vi "UHR-Fleezers Control (host) - Avogadro v2.vi"() -> ()   [LabVIEW 2014] (continued)
          tunnel: [FALSE w2222] -> w2201
          frame False {
          }
          frame True {
            n1371 = local read "Green FB On/Off"() -> (w2223:bool)
            n1372 = Equal?(x=w2226, y=enum32{"Laser ON", "Laser OFF", "Interlace"}."Interlace") -> (x = y?=w2224:bool)
            n1373 = And(x=w2224, y=w2223) -> (x .and. y?=w2222:bool)
          }
        }
        n1374 = case shown="True" "Red Laser ON" {
          tunnel: "Laser interlacing mode" -> [_ w2219]
          tunnel: [enum32{"Laser ON", "Laser OFF", "Interlace"}."Laser OFF" ("Green laser mode") w2219] -> w2198
          tunnel: [FALSE w2215] -> w2197
          frame False {
          }
          frame True {
            n1375 = local read "Red FB On/Off"() -> (w2216:bool)
            n1376 = Equal?(x=w2219, y=enum32{"Laser ON", "Laser OFF", "Interlace"}."Interlace") -> (x = y?=w2217:bool)
            n1377 = And(x=w2217, y=w2216) -> (x .and. y?=w2215:bool)
          }
        }
        n1378 = case shown="True" "Blue Laser ON" {
          tunnel: "Laser interlacing mode" -> [_ w2210]
          tunnel: [enum32{"Laser ON", "Laser OFF", "Interlace"}."Laser OFF" ("Green laser mode") w2210] -> w2194
          tunnel: [FALSE w2208] -> w2193
          frame False {
          }
          frame True {
            n1379 = local read "Blue FB On/Off"() -> (w2209:bool)
            n1380 = Equal?(x=w2210, y=enum32{"Laser ON", "Laser OFF", "Interlace"}."Interlace") -> (x = y?=w2211:bool)
            n1381 = And(x=w2211, y=w2209) -> (x .and. y?=w2208:bool)
          }
        }
        n1382 = xnode "Read/Write Control"("FPGA VI Reference In"=w2192, "Operating Mode"=w2202, "Operating Mode 2"=w2202, "Green FB On/Off"=w2201, "Red Laser Operating Mode"=w2198, "RI Operating Mode 2"=w2198, "Red FB On/Off"=w2197, "BI Operating Mode (AO)"=w2194, "Blue Laser Operating Mode (D)"=w2194, "Blue FB On/Off"=w2193) -> ("error out"=w2203:errorcluster)  [unwired: 1 in, 1 out]
        n1383 = local read "Red FB On/Off"() -> (w2175:bool)
        n1384 = local read "Green FB On/Off"() -> (w2177:bool)
        n1385 = local read "Green Laser ON"() -> (w2176:bool)
        n1386 = local read "Red Laser ON"() -> (w2174:bool)
        n1387 = And(x=w2175, y=w2174) -> (x .and. y?=w2180:bool)
        n1388 = And(x=w2177, y=w2176) -> (x .and. y?=w2186:bool)
        n1389 = local read "Red laser intensity (V)"() -> (w2179:dbl)
        n1390 = local read "Red FB Setpoint (mV)"() -> (w2178:dbl)
        n1391 = local read "Green FB Setpoint (mV)"() -> (w2189:dbl)
        n1392 = local read "Green laser intensity (V)"() -> (w2191:dbl)
        n1393 = Multiply(x=w2179, y=1000.0) -> (x*y=w2183:dbl)
        n1394 = Subtract(x=w2178, y=5.0) -> (x-y=w2182:dbl)
        n1395 = Multiply(x=w2191, y=1000.0) -> (x*y=w2188:dbl)
        n1396 = Subtract(x=w2189, y=5.0) -> (x-y=w2187:dbl)
        n1397 = Less Or Equal?(x=w2183, y=w2182) -> (x <= y?=w2181:bool)
        n1398 = Less Or Equal?(x=w2188, y=w2187) -> (x <= y?=w2185:bool)
        n1399 = And(x=w2180, y=w2181) -> (x .and. y?=w2170:bool)
        n1400 = And(x=w2186, y=w2185) -> (x .and. y?=w2171:bool)
        n1401 = Or(x=w2171, y=w2170) -> (x .or. y?=w2169:bool)
        n1402 = case shown="True" w2169 {
          frame False {
            n1403 = local write "Laser Intensity Low (bugs to fix)"(FALSE ("Laser Intensity Low")) -> ()
          }
          frame True {
            n1404 = local write "Laser Intensity Low (bugs to fix)"(TRUE ("Laser Intensity Low")) -> ()
          }
        }
      }
      event "Invert laser interlacing", "RF BD 2 to green AOM": Value Change {
        n1405 = event-data() -> ()  [unwired: 7 out]
        n1406 = local read "RF BD 2 to green AOM"() -> (w2227:bool)
        n1407 = xnode "Read/Write Control"("FPGA VI Reference In"=w2228, "Invert GI"="Invert laser interlacing", "Invert GI 2"="Invert laser interlacing", "Invert RI"="Invert laser interlacing", "Invert RI 2"="Invert laser interlacing", "Invert BI (AO)"="Invert laser interlacing", "Invert BI (D)"="Invert laser interlacing", "RF synth bd controls green"=w2227) -> ("error out"=w2230:errorcluster)  [unwired: 1 in, 1 out]
      }
      event "Green FB Setpoint (mV)", "Green FB Gains", "Green FB On/Off", "Green Intensity % (FB OFF)", "Green int current ON count adj": Value Change {
        n1408 = event-data() -> ()  [unwired: 7 out]
        n1409 = local read "Green FB Setpoint (mV)"() -> (w2250:dbl)
        n1410 = Multiply(x=w2250, y=3.2767) -> (x*y=w2249:dbl)
        n1411 = local read "Green Intensity % (FB OFF)"() -> (w2253:dbl)
        n1412 = Multiply(x=w2253, y=655.35) -> (x*y=w2254:dbl)
        n1413 = To Unsigned Word Integer(number=w2254) -> (unsigned 16bit integer=w2252:u16)
        n1414 = local read "Green int current ON count adj"() -> (w2256:u32)
        n1415 = local read "Laser interlacing mode"() -> (w2247:enum32{"Laser ON", "Laser OFF", "Interlace"})
        n1416 = local read "Green FB Gains"() -> (w2244:T18)
        n1417 = local read "Green Laser ON"() -> (w2248:bool)
        n1418 = local read "Green FB On/Off"() -> (w2257:bool)
        n1419 = Equal?(x=w2247, y=enum32{"Laser ON", "Laser OFF", "Interlace"}."Interlace") -> (x = y?=w2245:bool)
        n1420 = Unbundle By Name(w2244) -> ("proportional gain (Kc)"=w2243:i16, "integral gain (Kc*Ts/Ti)"=w2242:i16, "derivative gain (Kc*Td/Ts)"=w2241:i16)
        n1421 = Compound Arithmetic op=AND(w2245, w2257, w2248) -> (w2231:bool)
        n1422 = local read "Green FB Setpoint (mV)"() -> (w2235:dbl)
        n1423 = local read "Green laser intensity (V)"() -> (w2238:dbl)
        n1424 = xnode "Read/Write Control"("FPGA VI Reference In"=w2240, "Green FB Setpoint"=w2249, "Green FB On/Off"=w2231, "Current Out"=w2252, "Green int current ON count adj"=w2256, "P3"=w2243, "I3"=w2242, "D3"=w2241) -> ("error out"=w2258:errorcluster)  [unwired: 1 in, 1 out]
        n1425 = Multiply(x=w2238, y=1000.0) -> (x*y=w2234:dbl)
        n1426 = Subtract(x=w2235, y=5.0) -> (x-y=w2233:dbl)
        n1427 = Less Or Equal?(x=w2234, y=w2233) -> (x <= y?=w2232:bool)
        n1428 = And(x=w2231, y=w2232) -> (x .and. y?=w2239:bool)
        n1429 = case shown="True" w2239 {
          frame False {
            n1430 = local write "Laser Intensity Low (bugs to fix)"(FALSE ("Laser Intensity Low")) -> ()
          }
          frame True {
            n1431 = local write "Laser Intensity Low (bugs to fix)"(TRUE ("Laser Intensity Low")) -> ()
          }
        }
      }
      event "Blue FB Setpoint (mV)", "Blue FB Gains", "Blue FB On/Off", "Blue Intensity % (FB OFF)", "Blue int AO ON count adjust": Value Change {
        # "Triggers blue laser serial command"
        # "16 bit analog out"
        n1432 = event-data() -> ()  [unwired: 7 out]
        n1433 = Multiply(x="Blue FB Setpoint (mV)", y=3.2767) -> (x*y=w2278:dbl)
        n1434 = Multiply(x="Blue Intensity % (FB OFF)", y=0.8) -> (x*y=w2261:dbl)
        n1435 = Number To Decimal String(number=w2261) -> (decimal integer string=w2262:string)  [unwired: 1 in]
        n1436 = Multiply(x="Blue Intensity % (FB OFF)", y=655.35) -> (x*y=w2281:dbl)
        n1437 = local write "Blue Laser Power (mW)\n(Constant Power Mode)"(w2262) -> ()
        n1438 = To Unsigned Word Integer(number=w2281) -> (unsigned 16bit integer=w2280:u16)
        n1439 = local read "Laser interlacing mode"() -> (w2276:enum32{"Laser ON", "Laser OFF", "Interlace"})
        n1440 = Unbundle By Name("Blue FB Gains") -> ("proportional gain (Kc)"=w2273:i16, "integral gain (Kc*Ts/Ti)"=w2272:i16, "derivative gain (Kc*Td/Ts)"=w2271:i16)
        n1441 = local read "Blue Laser ON"() -> (w2266:bool)
        n1442 = Equal?(x=w2276, y=enum32{"Laser ON", "Laser OFF", "Interlace"}."Interlace") -> (x = y?=w2274:bool)
        n1443 = Compound Arithmetic op=AND(w2274, "Blue FB On/Off", w2266) -> (w2277:bool)
        n1444 = xnode "Read/Write Control"("FPGA VI Reference In"=w2265, "Blue FB Setpoint"=w2278, "Blue FB On/Off"=w2277, "BI Current Out"=w2280, "Blue current ON count adj (AO)"="Blue int AO ON count adjust", "P5"=w2273, "I5"=w2272, "D5"=w2271) -> ("error out"=w2283:errorcluster)  [unwired: 1 in, 1 out]
      }
      event "Red FB Setpoint (mV)", "Red FB Gains", "Red FB On/Off", "Red Intensity % (FB OFF)": Value Change {
        n1445 = event-data() -> ()  [unwired: 7 out]
        n1446 = local read "Red FB Setpoint (mV)"() -> (w2304:dbl)
        n1447 = Multiply(x=w2304, y=3.2767) -> (x*y=w2303:dbl)
        n1448 = local read "Red Intensity % (FB OFF)"() -> (w2294:dbl)
        n1449 = Multiply(x=w2294, y=655.35) -> (x*y=w2307:dbl)
        n1450 = To Unsigned Word Integer(number=w2307) -> (unsigned 16bit integer=w2306:u16)
        n1451 = local read "Laser interlacing mode"() -> (w2301:enum32{"Laser ON", "Laser OFF", "Interlace"})
        n1452 = local read "Red FB Gains"() -> (w2298:T18)
        n1453 = local read "Red Laser ON"() -> (w2302:bool)
        n1454 = local read "Red FB On/Off"() -> (w2309:bool)
        n1455 = Equal?(x=w2301, y=enum32{"Laser ON", "Laser OFF", "Interlace"}."Interlace") -> (x = y?=w2299:bool)
        n1456 = Unbundle By Name(w2298) -> ("proportional gain (Kc)"=w2297:i16, "integral gain (Kc*Ts/Ti)"=w2296:i16, "derivative gain (Kc*Td/Ts)"=w2295:i16)
        n1457 = Compound Arithmetic op=AND(w2299, w2309, w2302) -> (w2286:bool)
        n1458 = local read "Red laser intensity (V)"() -> (w2285:dbl)
        n1459 = local read "Red FB Setpoint (mV)"() -> (w2284:dbl)
        n1460 = xnode "Read/Write Control"("FPGA VI Reference In"=w2293, "Red FB Setpoint"=w2303, "Red FB On/Off"=w2286, "RI Current Out"=w2306, "P4"=w2297, "I4"=w2296, "D4"=w2295) -> ("error out"=w2310:errorcluster)  [unwired: 1 in, 1 out]
        n1461 = Multiply(x=w2285, y=1000.0) -> (x*y=w2290:dbl)
        n1462 = Subtract(x=w2284, y=5.0) -> (x-y=w2289:dbl)
        n1463 = Less Or Equal?(x=w2290, y=w2289) -> (x <= y?=w2288:bool)
        n1464 = And(x=w2286, y=w2288) -> (x .and. y?=w2287:bool)
        n1465 = case shown="False" w2287 {
          frame False {
            n1466 = local write "Laser Intensity Low (bugs to fix)"(FALSE ("Laser Intensity Low")) -> ()
          }
          frame True {
            n1467 = local write "Laser Intensity Low (bugs to fix)"(TRUE ("Laser Intensity Low")) -> ()
          }
        }
      }
      event "+ phase (APD 1 Gate)", "- phase (APD 1 Gate)", "+ phase (APD 2 Gate)", "- phase (APD 2 Gate)", "+ phase (APD 3 Gate)", "- phase (APD 3 Gate)", "+ phase (APD Acq)", "- phase (APD Acq)": Value Change {
        n1468 = event-data() -> ()  [unwired: 7 out]
        n1469 = local read "Phase Adj. (APD 1 Gate)"() -> (w2333:i16)
        n1470 = Or(x="- phase (APD 1 Gate)", y="+ phase (APD 1 Gate)") -> (x .or. y?=w2335:bool)
        n1471 = Negate(x=w2333) -> (-x=w2340:i16)
        n1472 = Select(t=w2340, s="+ phase (APD 1 Gate)", f=w2333) -> (s? t:f=w2339:i16)
        n1473 = local read "Phase Adj. (APD 2 Gate)"() -> (w2330:i16)
        n1474 = Or(x="- phase (APD 2 Gate)", y="+ phase (APD 2 Gate)") -> (x .or. y?=w2328:bool)
        n1475 = Negate(x=w2330) -> (-x=w2332:i16)
        n1476 = Select(t=w2332, s="+ phase (APD 2 Gate)", f=w2330) -> (s? t:f=w2329:i16)
        n1477 = Negate(x="Phase Adj. (APD 3 Gate)") -> (-x=w2327:i16)
        n1478 = Or(x="- phase (APD 3 Gate)", y="+ phase (APD 3 Gate)") -> (x .or. y?=w2323:bool)
        n1479 = Select(t=w2327, s="+ phase (APD 3 Gate)", f="Phase Adj. (APD 3 Gate)") -> (s? t:f=w2324:i16)
        n1480 = local read "Phase Adj. (APD Acq)"() -> (w2321:i16)
        n1481 = Or(x="- phase (APD Acq)", y="+ phase (APD Acq)") -> (x .or. y?=w2319:bool)
        n1482 = Negate(x=w2321) -> (-x=w2322:i16)
        n1483 = Select(t=w2322, s="+ phase (APD Acq)", f=w2321) -> (s? t:f=w2320:i16)
        n1484 = xnode "Read/Write Control"("FPGA VI Reference In"=w2313, "Phase count adjustment (APD 1 Gate)"=w2339, "Phase count adjustment (APD 2 Gate)"=w2329, "Phase count adjustment (APD 3 Gate)"=w2324, "Phase Count Adjustment (APD Acq)"=w2320) -> ("FPGA VI Reference Out"=w2337:T40, "error out"=w2338:errorcluster)  [unwired: 1 in]
        n1485 = xnode "Read/Write Control"("FPGA VI Reference In"=w2337, "error in"=w2338, "+ phase (APD 1 Gate)"=w2335, "+ phase (APD 2 Gate)"=w2328, "+ phase (APD 3 Gate)"=w2323, "+ phase (APD Acq)"=w2319) -> ("error out"=w2336:errorcluster)  [unwired: 1 out]
      }
      event "Invert APD Gate", "APD Gate ON Count", "APD Gate OFF Count", "APD Gate", "APD Integration Time (s)", "APD AO Scale Factor", "Duty Frequency (ON 1/N cycles)", "Interlace ON count", "Interlace OFF count": Value Change {
        n1486 = event-data() -> ()  [unwired: 7 out]
        n1487 = Add(x="Interlace ON count", y="Interlace OFF count") -> (x+y=w2347:u16)
        n1488 = Add(x="APD Gate ON Count", y="APD Gate OFF Count") -> (x+y=w2358:u16)
        n1489 = Multiply(x="Duty Frequency (ON 1/N cycles)", y=w2347) -> (x*y=w2343:u16)
        "Green AI Count" <- w2343
        "Red AI Count" <- w2343
        "Blue AI Count" <- w2343
        n1490 = Subtract(x=w2343, y="Interlace ON count") -> (x-y=w2346:u16)
        n1491 = Multiply(x=w2358, y="Duty Frequency (ON 1/N cycles)") -> (x*y=w2357:u16)
        n1492 = Subtract(x=w2357, y="APD Gate ON Count") -> (x-y=w2356:u16)
        n1493 = local read "DMA Update Period (s)"() -> (w2359:dbl)
        n1494 = Multiply(x="APD Integration Time (s)", y=40000000.0) -> (x*y=w2363:dbl)
        n1495 = Reciprocal(x="APD Integration Time (s)") -> (1/x=→"APD Acq Rate (Hz)":dbl)
        n1496 = To Unsigned Long Integer(number=w2363) -> (unsigned 32bit integer=w2349:u32)
        "APD Int. Count" <- w2349
        n1497 = local read "Number of APDs"() -> (w2342:u8)
        n1498 = Divide(x=w2359, y="APD Integration Time (s)") -> (x/y=w2361:dbl)
        n1499 = Multiply(x=w2342, y=w2361) -> (x*y=w2360:dbl)
        n1500 = local write "APD Samples/FIFO Acq."(w2361) -> ()
        n1501 = local write "APD Elements/DMA read"(w2360) -> ()
        n1502 = xnode "Read/Write Control"("FPGA VI Reference In"=w2341, "Invert APD Gate"="Invert APD Gate", "APD Gate ON Count"="APD Gate ON Count", "APD Gate OFF Count"=w2356, "APD Acq Rate Count"=w2349, "APD Gate Operating Mode"="APD Gate", "APD AO scale factor"="APD AO Scale Factor", "Green interlace ON count 2"="Interlace ON count", "Green interlace OFF count 2"=w2346, "Green FB Count"=w2343, "Red interlace ON count"="Interlace ON count", "Red interlace OFF count"="Interlace OFF count", "Blue ON count (AO)"="Interlace ON count", "Blue OFF count (AO)"="Interlace OFF count", "Blue interlace OFF count (D)"="Interlace OFF count", "Blue interlace ON count (D)"="Interlace ON count") -> ("error out"=w2365:errorcluster)  [unwired: 1 in, 1 out]
      }
      event "Neg. TTrig FPGA": Value Change {
        n1503 = event-data() -> ()  [unwired: 7 out]
        n1504 = xnode "Read/Write Control"("FPGA VI Reference In"=w2366, "TTrig Negate Pos"="Neg. TTrig FPGA") -> ()  [unwired: 1 in, 2 out]
      }
      event "Test ttrig": Value Change {
        n1505 = event-data() -> ()  [unwired: 7 out]
        n1506 = xnode "Read/Write Control"("FPGA VI Reference In"=w2368, "TTrig?"=TRUE) -> ("error out"=w2370:errorcluster)  [unwired: 1 in, 1 out]
      }
      event "Number of F/B Scans (AOD)", "Scan Speed (nm/s)", "Scan BD", "Initial delta (MHz)", "Step Size (nm)", "Scan Range (nm)": Value Change {
        w2434 = 123.0  # AOM cal (nm/MHz)
        n1507 = event-data() -> ()  [unwired: 7 out]
        n1508 = local read "BD 1 Frequency 1 (MHz)"() -> (w2417:dbl)
        n1509 = local read "AOM X Cal (nm/MHz)"() -> (w2409:dbl)
        n1510 = local read "X RF Frequency Limits (MHz)"() -> (w2421:T26)
        n1511 = local read "Y RF Frequency Limits (MHz)"() -> (w2418:T26)
        n1512 = local read "BD 2 Frequency 1 (MHz)"() -> (w2423:dbl)
        n1513 = Negate(x="Scan Range (nm)") -> (-x=w2387:dbl)
        n1514 = Divide(x=w2387, y=w2409) -> (x/y=w2391:dbl)
        n1515 = Select(t=w2421, s="Scan BD", f=w2418) -> (s? t:f=w2420:T26)
        n1516 = Select(t=w2417, s="Scan BD", f=w2423) -> (s? t:f=w2422:dbl)
        n1517 = Unbundle By Name(w2420) -> ("Maximum"=w2429:dbl, "Minimum"=w2428:dbl)
        n1518 = Add(x=w2391, y=w2422) -> (x+y=w2426:dbl)
        n1519 = Divide(x=w2387, y="Step Size (nm)") -> (x/y=w2406:dbl)
        n1520 = Divide(x="Step Size (nm)", y=w2409) -> (x/y=w2415:dbl)
        n1521 = Absolute Value(x=w2406) -> (abs(x)=w2390:dbl)
        n1522 = Sign(1:w2387) -> (0:w2388:dbl)
        n1523 = In Range and Coerce(upper limit=w2429, x=w2426, lower limit=w2428) -> (coerced(x)=w2425:dbl, In Range?=w2427:bool)
        n1524 = To Unsigned Quad Integer(1:w2390) -> (0:w2405:u64)
        "Scan steps (AOD)" <- w2405
        n1525 = call "IR AOM freq to word.vi"("Frequency In (MHz)"=w2415) -> ("Frequency Word Out (double)"=w2412:dbl)
        n1526 = Multiply(x=w2388, y=w2412) -> (x*y=w2389:dbl)
        n1527 = Subtract(x=w2426, y=w2425) -> (x-y=w2424:dbl)
        n1528 = To Quad Integer(1:w2389) -> (0:w2411:i64)
        "Incr. int (AOD)" <- w2411
        n1529 = Subtract(x=w2391, y=w2424) -> (x-y=w2410:dbl)
        "Scan Range (MHz)" <- w2410
        n1530 = Select(t=w2391, s=w2427, f=w2410) -> (s? t:f=w2430:dbl)
        n1531 = Multiply(x=w2410, y=w2409) -> (x*y=w2408:dbl)
        n1532 = Decrement(x=w2405) -> (x-1=w2458:u64)
        n1533 = Negate(x=w2408) -> (-x=w2404:dbl)
        n1534 = local write "Scan Range (nm)"(w2404) -> ()
        n1535 = Divide(x=w2430, y=w2458) -> (x/y=w2414:dbl)
        "Scan Increment (MHz)" <- w2414
        n1536 = call "IR AOM freq to word.vi"("Frequency In (MHz)"=w2414) -> ("Frequency Word Out (double)"=w2413:dbl)
        n1537 = Divide(x="Step Size (nm)", y="Scan Speed (nm/s)") -> (x/y=w2401:dbl)
        n1538 = To Quad Integer(1:w2413) -> ()  [unwired: 1 out]
        n1539 = local read "Number Interlace Sets"() -> (w2385:u8)
        n1540 = local read "AI Count (ticks)"() -> (w2386:u16)
        n1541 = local read "Total Counts (ticks)"() -> (w2384:u16)
        n1542 = local read "# Samples/trap"() -> (w2416:u32)
        n1543 = Multiply(x=w2386, y=w2385) -> (x*y=w2383:u16)
        n1544 = Divide(x=w2384, y=w2383) -> (x/y=w2382:dbl)
        n1545 = Select(t=w2417, s="Scan BD", f=w2423) -> (s? t:f=w2455:dbl)
        "Initial freq. (MHz)" <- w2455
        n1546 = Add(x=w2430, y=w2455) -> (x+y=→"Final freq. (MHz)":dbl)
        n1547 = Divide(x=w2384, y=40000000.0) -> (x/y=w2400:dbl)
        n1548 = Divide(x=w2401, y=w2400) -> (x/y=w2399:dbl)
        n1549 = To Unsigned Quad Integer(1:w2399) -> (0:w2374:u64)
        n1550 = Quotient & Remainder(x=w2374, y=u64 2) -> (x-y*floor(x/y)=w2378:u64)  [unwired: 1 out]
        n1551 = Equal?(x=w2378, y=u64 0) -> (x = y?=w2376:bool)
        n1552 = Decrement(x=w2374) -> (x-1=w2375:u64)
        n1553 = Select(t=w2374, s=w2376, f=w2375) -> (s? t:f=w2373:u64)
        "Cycles/step (AOD)" <- w2373
        n1554 = xnode "Read/Write Control"("FPGA VI Reference In"=w2372, "Scan steps"=w2405, "Number of scans"="Number of F/B Scans (AOD)", "Cycles per step"=w2373, "Scan freq.  increment"=w2411, "Scan BD"="Scan BD") -> ("error out"=w2464:errorcluster)  [unwired: 1 in, 1 out]
        n1555 = Multiply(x=w2405, y=w2373) -> (x*y=w2459:u64)
        n1556 = Multiply(x=w2459, y=u64 2) -> (x*y=w2381:u64)
        n1557 = Multiply(x=w2382, y=w2381) -> (x*y=w2380:dbl)
        "Data points/scan (f/b)" <- w2380
        n1558 = Multiply(x=w2380, y="Number of F/B Scans (AOD)") -> (x*y=w2462:dbl)
        "Data points/scans" <- w2462
        n1559 = Divide(x=w2462, y=w2416) -> (x/y=→"N sets should be saved":dbl)
        n1560 = Multiply(x=w2459, y=w2400) -> (x*y=w2398:dbl)
        "Time/Scan (s) (AOD)" <- w2398
        n1561 = Select(t=w2430, s="Scan BD", f=0.0) -> (s? t:f=w2456:dbl)
        n1562 = Select(t=0.0, s="Scan BD", f=w2430) -> (s? t:f=w2452:dbl)
        n1563 = local read "BD 2 Frequency 2 (MHz)"() -> (w2448:dbl)
        n1564 = local read "BD 1 Frequency 2 (MHz)"() -> (w2451:dbl)
        n1565 = Add(x=w2452, y=w2423) -> (x+y=w2449:dbl)
        n1566 = Add(x=w2417, y=w2456) -> (x+y=w2450:dbl)
        n1567 = Multiply(x=w2398, y=2.0) -> (x*y=w2397:dbl)
        n1568 = Multiply(x=w2397, y="Number of F/B Scans (AOD)") -> (x*y=w2394:dbl)
        n1569 = Divide(x=w2394, y=60.0) -> (x/y=→"Time to Finish All (min)":dbl)
        n1570 = Add(x="Trap 2 Bead Size (nm)", y="Trap 1 Bead Size (nm)") -> (x+y=w2438:dbl)
        n1571 = Divide(x=w2438, y=2.0) -> (x/y=w2432:dbl)
        n1572 = local read "Initial delta (MHz)"() -> (w2435:dbl)
        n1573 = Subtract(x=w2449, y=w2448) -> (x-y=w2446:dbl)
        n1574 = Subtract(x=w2450, y=w2451) -> (x-y=w2447:dbl)
        n1575 = Square(x=w2446) -> (x^2=w2445:dbl)
        n1576 = Square(x=w2447) -> (x^2=w2444:dbl)
        n1577 = Add(x=w2444, y=w2445) -> (x+y=w2443:dbl)
        n1578 = Square Root(x=w2443) -> (sqrt(x)=w2442:dbl)
        "Final delta (MHz)" <- w2442
        n1579 = Multiply(x=w2434, y=w2442) -> (x*y=w2441:dbl)
        n1580 = Multiply(x=w2435, y=w2434) -> (x*y=w2433:dbl)
        n1581 = Subtract(x=w2433, y=w2432) -> (x-y=→"Initial sep (nm)":dbl)
        n1582 = Subtract(x=w2441, y=w2432) -> (x-y=→"Final sep (nm)":dbl)
      }
      event "Swap F1 and F2", "RF amplitude switch delay": Value Change {
        n1583 = event-data() -> ()  [unwired: 7 out]
        n1584 = local read "RF amplitude switch delay"() -> (w2466:u16)
        n1585 = local read "Swap F1 and F2"() -> (w2467:bool)
        n1586 = xnode "Read/Write Control"("FPGA VI Reference In"=w2465, "Swap F1 and F2"=w2467, "Amp switch delay"=w2466) -> ("error out"=w2468:errorcluster)  [unwired: 1 in, 1 out]
      }
      event "Scan steps (MCL)", "Number of scans (MCL)", "Scan Range (V)\n(of steps)", "2D or 1D Scan", "N APD Samp/step", "Fast Scan Dir", "Continuous MCL Scanning", "Scan lines (y)": Value Change {
        w2471 = 32767.0 ("y")
        n1587 = event-data() -> ()  [unwired: 7 out]
        n1588 = Select(t="Scan lines (y)", s="2D or 1D Scan", f="Number of scans (MCL)") -> (s? t:f=w2476:u64)
        n1589 = Decrement(x="Scan steps (MCL)") -> (x-1=w2492:u64)
        n1590 = Divide(x="Scan Range (V)\n(of steps)", y=w2492) -> (x/y=w2491:dbl)
        "Desired Scan Incr (V)" <- w2491
        n1591 = local read "APD Integration Time (s)"() -> (w2484:dbl)
        n1592 = Multiply(x=w2491, y=w2471) -> (x*y=w2500:dbl)
        n1593 = Divide(x=w2500, y=10.0) -> (x/y=w2490:dbl)
        "Desired incr (int)" <- w2490
        n1594 = local read "Update Count (MCL)"() -> (w2496:u32)
        n1595 = Round Toward -Infinity(1:w2490) -> (0:w2499:dbl)
        n1596 = To Word Integer(number=w2499) -> (16bit integer=w2474:i16)
        "Actual Incr. int (MCL)" <- w2474
        n1597 = Multiply(x=w2484, y=40000000.0) -> (x*y=w2497:dbl)
        n1598 = Divide(x=w2497, y=w2496) -> (x/y=w2495:dbl)
        n1599 = Multiply(x=i16 10, y=w2474) -> (x*y=w2472:i16)
        n1600 = Multiply(x="N APD Samp/step", y=w2495) -> (x*y=w2494:dbl)
        "Cycles/step (MCL)" <- w2494
        n1601 = Divide(x=w2472, y=w2471) -> (x/y=→"Actual MCL Inc (V)":dbl)
        n1602 = Multiply(x="N APD Samp/step", y="Scan steps (MCL)") -> (x*y=w2486:dbl)
        n1603 = local read "APD Samples/FIFO Acq."() -> (w2483:dbl)
        n1604 = Multiply(x=w2486, y=u64 2) -> (x*y=w2485:dbl)
        "Data points/scan (f+b)" <- w2485
        n1605 = Multiply(x=w2485, y=w2476) -> (x*y=w2503:dbl)
        "Data points/scans (MCL)" <- w2503
        n1606 = Multiply(x=w2484, y=w2485) -> (x*y=w2477:dbl)
        "Time/f+b scan (s) (MCL)" <- w2477
        n1607 = Divide(x=w2503, y=w2483) -> (x/y=→"N sets should be saved (MCL)":dbl)
        n1608 = Multiply(x=w2477, y=w2476) -> (x*y=→"Total Time (s)":dbl)
        n1609 = Not(x="Fast Scan Dir") -> (.not. x?=w2481:bool)
        n1610 = xnode "Read/Write Control"("FPGA VI Reference In"=w2469, "Scan steps (MCL)"="Scan steps (MCL)", "Number of scans (MCL)"=w2476, "Cycles per step (MCL)"=w2494, "Scan freq.  increment (MCL)"=w2474, "1D or 2D Scan?"="2D or 1D Scan", "MCL Scan Axis"=w2481, "Cont. Scan (MCL)"="Continuous MCL Scanning") -> ("error out"=w2505:errorcluster)  [unwired: 1 in, 1 out]
      }
      event "Read Cal": Value Change {
        w2528 = T53."big-endian, network order" ("byte order (0:big-endian, network order)")
        n1611 = event-data() -> ()  [unwired: 7 out]
        n1612 = local read "Save file name"() -> (w2553:path)
        n1613 = Strip Path(path=w2553) -> (stripped path=w2552:path)  [unwired: 1 out]
        n1614 = Path To String(path=w2552) -> (string=w2545:string)
        n1615 = Concatenate Strings(w2545, "\\current.cal" ("string")) -> (w2550:string)
        n1616 = String To Path(string=w2550) -> (path=w2549:path)
        n1617 = Concatenate Strings(w2545, "\\current.off" ("string")) -> (w2543:string)
        n1618 = Open/Create/Replace File(file path (use dialog)=w2549, operation (0:open)=T52."open", access (0:read/write)=enum16{"read/write", "read-only", "write-only"}."read-only") -> (refnum out=w2556:refnum<file>, error out=w2548:errorcluster)  [unwired: 1 in, 3 out]
        n1619 = Deny Access(4:w2548, 7:w2556) -> (0:w2529:errorcluster, 3:w2524:refnum<file>)  [unwired: 1 out]
        n1620 = String To Path(string=w2543) -> (path=w2540:path)
        n1621 = local write "Read Cal"(FALSE ("Read Cal")) -> ()
        n1622 = Open/Create/Replace File(file path (use dialog)=w2540, operation (0:open)=T52."open", access (0:read/write)=enum16{"read/write", "read-only", "write-only"}."read-only") -> (refnum out=w2539:refnum<file>)  [unwired: 1 in, 4 out]
        n1623 = Deny Access(7:w2539) -> (3:w2538:refnum<file>)  [unwired: 1 in, 2 out]
        n1624 = Read from Binary File(5:0.0, 9:w2528, 10:-1 ("count (1)"), 11:w2538) -> (2:w2506:dbl[], 3:w2535:refnum<file>)  [unwired: 1 in, 3 out]
        "Raw offsets" <- w2506
        n1625 = local read "Multiple-MCL offset?"() -> (w2507:bool)
        n1626 = Close File(refnum=w2535) -> ()  [unwired: 1 in, 2 out]
        n1627 = case shown="True" w2507 {
          tunnel: w2506 -> [w2561 w2568]
          tunnel: [w2558 w2566] -> w2533
          tunnel: [w2557 w2565] -> w2532
          frame False {
            # "If not doing multiple offset, same calculation as before"
            n1628 = Decimate 1D Array(w2561) -> (w2558:dbl[], w2557:dbl[])
            n1629 = Bundle By Name(cluster="Two Trap Offset Values", "Trap 1X offset"=w2558, "Trap 2X offset"=w2557) -> (w2559:T31)
            n1630 = local write "Two Trap Offset Values"(w2559) -> ()
          }
          frame True {
            w2563 = 0.0
            # "When doing multiple offset: separate data to different scans, make array of clusters of 1x,1y,2x,2y,3x,3y arrays"
            n1631 = local read "MCL offset scanning range (V)"() -> (w2569:T4)
            n1632 = local read "Offset file step size"() -> (w2567:dbl)
            n1633 = Build Array(w2563, w2563, w2563, w2563, w2563, w2563) -> (w2562:dbl[])
            n1634 = call "generate multiple MCL offset.vi"("Offset array"=w2568, "offset file step size"=w2567, "MCL offset scanning range (V)"=w2569, "Corrections"=w2562) -> ("B_X mean out"=w2565:dbl[], "A_X mean out"=w2566:dbl[], "Output array"=→"Multi-MCL offset array":T30)
          }
        }
        n1635 = Build Array("T1 calibration", "T2 calibration", "T3 calibration") -> (w2520:T55)
        n1636 = for {
          N: 3 ("count (1)") -> [_]
          tunnel: w2528 -> [w2587]
          shift-right: [w2585] -> w2526
          shift-left: w2529 -> [w2588]
          shift-right: [w2584] -> w2525
          shift-left: w2524 -> [w2583]
          tunnel: w2520 -> [w2582] mode=indexing
          tunnel: [w2576] -> w2519 mode=indexing
          i -> [w2577]
          w2571 = 1000.0
          n1637 = Read from Binary File(5:0.0, 8:w2588, 9:w2587, 10:6 ("count (1)"), 11:w2583) -> (0:w2585:errorcluster, 2:w2590:dbl[], 3:w2584:refnum<file>)  [unwired: 2 out]
          n1638 = Array To Cluster(array=w2590) -> (cluster=w2581:T56)
          n1639 = Unbundle(w2581) -> ("[0]"=w2580:dbl, "[1]"=w2579:dbl, "[2]"=w2573:dbl, "[3]"=w2578:dbl, "[4]"=w2572:dbl, "[5]"=w2575:dbl)
          n1640 = Multiply(x=w2572, y=w2571) -> (x*y=w2570:dbl)
          n1641 = Multiply(x=w2571, y=w2575) -> (x*y=w2574:dbl)
          n1642 = Bundle By Name(cluster=w2582, "alpha_x (nm/V)"=w2580, "alpha_y (nm/V)"=w2579, "kappa_x (pN/nm)"=w2573, "kappa_y (pN/nm)"=w2578, "offset_x (mV)"=w2570, "offset_y (mV)"=w2574) -> (w2576:T12)
          n1643 = case shown="2" w2577 {
            tunnel: w2576 -> [w2591 w2592 w2593]
            frame 0, Default {
              n1644 = local write "T1 calibration"(w2591) -> ()
            }
            frame 1 {
              n1645 = local write "T2 calibration"(w2592) -> ()
            }
            frame 2 {
              n1646 = local write "T3 calibration"(w2593) -> ()
            }
          }
        }
        n1647 = Index Array(array=w2519, index=1) -> (element=w2516:T12)
        n1648 = Index Array(array=w2519, index=0) -> (element=w2515:T12)
        n1649 = Unbundle By Name(w2516) -> ("alpha_x (nm/V)"=w2514:dbl, "kappa_x (pN/nm)"=w2513:dbl)
        n1650 = Unbundle By Name(w2515) -> ("alpha_x (nm/V)"=w2512:dbl, "kappa_x (pN/nm)"=w2511:dbl)
        n1651 = Close File(refnum=w2525, error in=w2526) -> (error out=→"Read cal error":errorcluster)  [unwired: 1 out]
        n1652 = Multiply(x=w2514, y=w2513) -> (x*y=w2510:dbl)
        n1653 = Multiply(x=w2512, y=w2511) -> (x*y=w2509:dbl)
        n1654 = Divide(x=w2510, y=w2509) -> (x/y=w2508:dbl)
        n1655 = property on="B factor" class="DigNum (strict)"("Val(Sgnl)"=w2508) -> ()  [unwired: 2 in, 2 out]
        n1656 = Multiply(x=w2532, y=w2508) -> (x*y=w2534:dbl[])
        n1657 = Subtract(x=w2533, y=w2534) -> (x-y=w2530:dbl[])
        n1658 = case shown="True" "Auto read offset correction" {
          tunnel: w2530 -> [_ w2594]
          frame False {
          }
          frame True {
            n1659 = property on="Setpoint offset\ncorrection values" class="Arr (strict)"("Val(Sgnl)"=w2594) -> ()  [unwired: 2 in, 2 out]
          }
        }
      }
      event "Abort MCL Scan": Value Change {
        n1660 = event-data() -> ()  [unwired: 7 out]
        n1661 = local write "MCL Scanning"(FALSE ("MCL Scanning")) -> ()
        n1662 = xnode "Read/Write Control"("FPGA VI Reference In"=w2595, "Abort scan (MCL)"="Abort MCL Scan") -> ("error out"=w2598:errorcluster)  [unwired: 1 in, 1 out]
      }
      event "Update Count (MCL)": Value Change {
        n1663 = event-data() -> ()  [unwired: 7 out]
        n1664 = xnode "Read/Write Control"("FPGA VI Reference In"=w2599, "MCL count"="Update Count (MCL)") -> ("error out"=w2601:errorcluster)  [unwired: 1 in, 1 out]
      }
      event "+ phase (MCL)", "- phase (MCL)": Value Change {
        n1665 = event-data() -> ()  [unwired: 7 out]
        n1666 = Or(x="- phase (MCL)", y="+ phase (MCL)") -> (x .or. y?=w2605:bool)
        n1667 = Negate(x="Phase adjust (MCL)") -> (-x=w2611:i16)
        n1668 = Select(t=w2611, s="+ phase (MCL)", f="Phase adjust (MCL)") -> (s? t:f=w2609:i16)
        n1669 = xnode "Read/Write Control"("FPGA VI Reference In"=w2602, "Phase count adjustment (MCL)"=w2609) -> ("FPGA VI Reference Out"=w2606:T40, "error out"=w2607:errorcluster)  [unwired: 1 in]
        n1670 = xnode "Read/Write Control"("FPGA VI Reference In"=w2606, "error in"=w2607, "+ phase (MCL)"=w2605) -> ("error out"=w2604:errorcluster)  [unwired: 1 out]
      }
      event "Abort AOD Scan": Value Change {
        n1671 = event-data() -> ()  [unwired: 7 out]
        n1672 = xnode "Read/Write Control"("FPGA VI Reference In"=w2612, "Abort scan"="Abort AOD Scan") -> ("error out"=w2614:errorcluster)  [unwired: 1 in, 1 out]
      }
      event "Continuous AOD Scanning": Value Change {
        n1673 = event-data() -> ()  [unwired: 7 out]
        n1674 = xnode "Read/Write Control"("FPGA VI Reference In"=w2615, "Cont. Scan"="Continuous AOD Scanning") -> ("error out"=w2617:errorcluster)  [unwired: 1 in, 1 out]
      }
      event "Index": Value Change {
        n1675 = event-data() -> ()  [unwired: 7 out]
        n1676 = call "Create new save file.vi"("Insert"="", "Ext"=".dat" ("string"), "Index In"="Index") -> ("Path Out"=→"Save file name":path, "Index Out"=w2618:dbl)
        "Save index" <- w2618
        n1677 = local write "Index"(w2618) -> ()
      }
      event "AO1", "AO2": Value Change {
        w2632 = 10.0 ("y")
        w2631 = 32767.0 ("y")
        n1678 = event-data() -> ()  [unwired: 7 out]
        n1679 = local read "AO2"() -> (w2630:dbl)
        n1680 = local read "AO1"() -> (w2627:dbl)
        n1681 = Multiply(x=w2627, y=w2631) -> (x*y=w2626:dbl)
        n1682 = Multiply(x=w2630, y=w2631) -> (x*y=w2629:dbl)
        n1683 = Divide(x=w2626, y=w2632) -> (x/y=w2625:dbl)
        n1684 = Divide(x=w2629, y=w2632) -> (x/y=w2628:dbl)
        n1685 = To Word Integer(number=w2625) -> (16bit integer=w2633:i16)
        n1686 = To Word Integer(number=w2628) -> (16bit integer=w2634:i16)
        n1687 = xnode "Read/Write Control"("FPGA VI Reference In"=w2623, "AO1 (Y)"=w2633, "AO2 (X)"=w2634) -> ("error out"=w2624:errorcluster)  [unwired: 1 in, 1 out]
      }
      event "Inject Pump 1": Value Change {
        n1688 = event-data() -> ()  [unwired: 7 out]
        n1689 = disable-structure shown="Disabled" {
          disable-tunnel: w2635 -> [w2636 _]
          frame Disabled {
            n1690 = local read "Use Harvard pumps\nfor beads (else Chemyx)"() -> (w2637:bool)
            n1691 = case shown="True" w2637 {
              tunnel: "Inject Pump 1" -> [w2641 w2682]
              tunnel: w2636 -> [_ w2683]
              frame False {
                n1692 = local read "Pump write delay (ms)"() -> (w2640:dbl)
                n1693 = local read "Chemyx Syringe Pump Serial Port"() -> (w2639:refnum<visa-resource-name>)
                n1694 = case shown="True" w2641 {
                  tunnel: w2640 -> [w2647 w2661]
                  tunnel: w2639 -> [w2644 w2660]
                  frame False {
                    n1695 = flat-sequence {
                      tunnel: w2644 -> [w2648]
                      tunnel: [w2648] -> w2645
                      tunnel: w2647 -> [_]
                      tunnel: [w2651] -> w2646
                      tunnel: w2645 -> [w2651]
                      tunnel: w2646 -> [w2652]
                      tunnel: [w2652] -> w2642
                      tunnel: [w2654] -> w2643
                      tunnel: w2642 -> [w2654]
                      tunnel: w2643 -> [w2656]
                      frame #0 {
                        n1696 = call "Write to pump.vi"("string"="enter pump1", "VISA resource name"=w2648) -> ()  [unwired: 1 out]
                      }
                      frame #1 {
                        n1697 = Wait (ms)(milliseconds to wait="Pump pause delay (ms)") -> ()  [unwired: 1 out]
                      }
                      frame #2 {
                        n1698 = call "Write to pump.vi"("string"="stop", "VISA resource name"=w2652) -> ()  [unwired: 1 out]
                      }
                      frame #3 {
                        n1699 = Wait (ms)(milliseconds to wait=u32 500) -> ()  [unwired: 1 out]
                      }
                      frame #4 {
                        n1700 = call "Write to pump.vi"("string"="stop", "VISA resource name"=w2656) -> ()  [unwired: 1 out]
                      }
                    }
                  }
                  frame True {
                    n1701 = flat-sequence {
                      tunnel: w2660 -> [w2670]
                      tunnel: w2661 -> [w2665]
                      tunnel: w2661 -> [w2672]
                      tunnel: w2660 -> [w2673]
                      tunnel: [w2673] -> w2658
                      tunnel: [w2675] -> w2659
                      tunnel: w2658 -> [w2675]
                      tunnel: w2659 -> [w2677]
                      frame #0 {
                        n1702 = local read "All Pump Parameters"() -> (w2664:T14)
                        n1703 = Unbundle By Name(w2664) -> ("Pump 1"=w2671:T57)
                        n1704 = call "Set pump parameters.vi"("Pump write delay (ms)"=w2665, "Volume (uL)"="Ch 1 Inject Volume (uL)", "Rate (uL/h)"="Ch 1 Inject Rate (ul/h)", "Units"=4.0, "Pump #"=1.0, "Pump Parameters In"=w2671, "VISA resource name"=w2670) -> ("Pump Parameters Out"=w2663:T57)  [unwired: 3 in]
                        n1705 = Bundle By Name(cluster=w2664, "Pump 1"=w2663) -> (w2662:T14)
                        n1706 = local write "All Pump Parameters"(w2662) -> ()
                      }
                      frame #1 {
                        n1707 = Wait (ms)(milliseconds to wait=w2672) -> ()  [unwired: 1 out]
                      }
                      frame #2 {
                        n1708 = call "Write to pump.vi"("string"="start", "VISA resource name"=w2673) -> ()  [unwired: 1 out]
                      }
                      frame #3 {
                        n1709 = Wait (ms)(milliseconds to wait=u32 500) -> ()  [unwired: 1 out]
                      }
                      frame #4 {
                        n1710 = call "Write to pump.vi"("string"="start", "VISA resource name"=w2677) -> ()  [unwired: 1 out]
                      }
                    }
                  }
                }
              }
              frame True {
                n1711 = case shown="False" w2682 {
                  tunnel: w2683 -> [w2695 w2705]
                  frame False {
                    n1712 = flat-sequence {
                      tunnel: w2695 -> [w2697]
                      frame #0 {
                        n1713 = local write "Flushing P1"(FALSE ("Flushing P1")) -> ()
                        n1714 = Concatenate Strings("stop" ("string"), "\r") -> (w2699:string)
                        n1715 = VISA Write(VISA resource name=w2697, write buffer=w2699) -> ()  [unwired: 1 in, 3 out]
                      }
                      frame #1 {
                        n1716 = property on="Clear Volume P1" class="Bool (strict)"("Val(Sgnl)"=TRUE ("Value (Signaling)")) -> ()  [unwired: 2 in, 2 out]
                      }
                    }
                  }
                  frame True {
                    n1717 = local read "Normal Flow Rate (ul/h) P1"() -> (w2703:dbl)
                    n1718 = Number To Decimal String(number=w2703) -> (decimal integer string=w2709:string)  [unwired: 1 in]
                    n1719 = Concatenate Strings("irate  " ("string"), w2709, " u/h" ("string"), "\r") -> (w2707:string)
                    n1720 = VISA Write(VISA resource name=w2705, write buffer=w2707) -> (VISA resource name out=w2704:refnum<visa-resource-name>)  [unwired: 1 in, 2 out]
                    n1721 = Concatenate Strings("irun" ("string"), "\r") -> (w2711:string)
                    n1722 = VISA Write(VISA resource name=w2704, write buffer=w2711) -> ()  [unwired: 1 in, 3 out]
                  }
                }
                n1723 = local read "Saving..."() -> (w2680:bool)
                n1724 = local read "Save Event Log?"() -> (w2679:bool)
                n1725 = And(x=w2680, y=w2679) -> (x .and. y?=w2681:bool)
                n1726 = case shown="True" w2681 {
                  tunnel: w2682 -> [_ w2693]
                  frame False {
                  }
                  frame True {
                    n1727 = local read "Normal Flow Rate (ul/h) P1"() -> (w2684:dbl)
                    n1728 = Number To Decimal String(number=w2684) -> (decimal integer string=w2685:string)  [unwired: 1 in]
                    n1729 = Concatenate Strings("on, flow rate", w2685) -> (w2687:string)
                    n1730 = Select(t=w2687, s=w2693, f="off") -> (s? t:f=w2689:string)
                    n1731 = local read "log file ref"() -> (w2694:refnum<file>)
                    n1732 = local read "Time (s)"() -> (w2688:dbl)
                    n1733 = Concatenate Strings("pump 1 ", w2689) -> (w2691:string)
                    n1734 = call "write to event log.vi"("log file ref"=w2694, "time"=w2688, "input string"=w2691) -> ()  [unwired: 8 in]
                  }
                }
              }
            }
          }
          frame Enabled {
          }
        }
      }
      event "Shunt 1": Value Change {
        n1735 = event-data() -> ()  [unwired: 7 out]
        n1736 = local read "Visa resource for valves"() -> (w2713:refnum<visa-resource-name>)
        n1737 = call "hamilton_controller.vi"("VISA resource name in"=w2713, "Open?"="Shunt 1", "valve"=enum16{"A", "B", "ALL"}."A", "action"=T48."MOVE VALVE") -> ("error out"=w2715:errorcluster)  [unwired: 6 in, 1 out]
      }
      event "Shunt 2": Value Change {
        n1738 = event-data() -> ()  [unwired: 7 out]
        n1739 = case shown="True" "Shunt 2" {
          tunnel: [w2722 w2728] -> w2720
          tunnel: w2718 -> [_ w2726]
          frame False {
            n1740 = local read "Visa resource for valves"() -> (w2723:refnum<visa-resource-name>)
            n1741 = call "hamilton_controller.vi"("VISA resource name in"=w2723, "Open?"=FALSE, "valve"=enum16{"A", "B", "ALL"}."B", "action"=T48."MOVE VALVE") -> ("error out"=w2722:errorcluster)  [unwired: 6 in, 1 out]
          }
          frame True {
            n1742 = case shown="True" "Auto switch off shunt?" {
              tunnel: [w2731 w2742] -> w2728
              tunnel: w2726 -> [_ w2735]
              frame False {
                n1743 = local read "Visa resource for valves"() -> (w2730:refnum<visa-resource-name>)
                n1744 = call "hamilton_controller.vi"("VISA resource name in"=w2730, "Open?"=TRUE, "valve"=enum16{"A", "B", "ALL"}."B", "action"=T48."MOVE VALVE") -> ("error out"=w2731:errorcluster)  [unwired: 6 in, 1 out]
              }
              frame True {
                n1745 = flat-sequence {
                  tunnel: [w2746] -> w2743
                  tunnel: [w2745] -> w2736
                  tunnel: w2735 -> [w2745]
                  tunnel: [w2752] -> w2744
                  tunnel: w2743 -> [w2752]
                  tunnel: [w2751] -> w2737
                  tunnel: w2736 -> [w2751]
                  tunnel: w2744 -> [w2758]
                  tunnel: [w2757] -> w2740
                  tunnel: [w2756] -> w2738
                  tunnel: w2737 -> [w2756]
                  tunnel: [w2764] -> w2741
                  tunnel: w2740 -> [w2764]
                  tunnel: [w2763] -> w2739
                  tunnel: w2738 -> [w2763]
                  tunnel: w2741 -> [w2767]
                  tunnel: w2739 -> [w2766]
                  tunnel: [w2767] -> w2734
                  tunnel: [w2772] -> w2742
                  tunnel: w2734 -> [w2772]
                  frame #0 {
                    n1746 = local read "Visa resource for valves"() -> (w2748:refnum<visa-resource-name>)
                    n1747 = call "hamilton_controller.vi"("VISA resource name in"=w2748, "Open?"=TRUE, "valve"=enum16{"A", "B", "ALL"}."B", "action"=T48."MOVE VALVE") -> ("error out"=w2746:errorcluster)  [unwired: 6 in, 1 out]
                  }
                  frame #1 {
                    n1748 = Multiply(x="Shunt switch off time (s)", y=1000) -> (x*y=w2753:i32)
                    n1749 = Wait (ms)(milliseconds to wait=w2753) -> ()  [unwired: 1 out]
                  }
                  frame #2 {
                    n1750 = local read "Visa resource for valves"() -> (w2761:refnum<visa-resource-name>)
                    n1751 = call "hamilton_controller.vi"("VISA resource name in"=w2761, "error in"=w2758, "Open?"=FALSE, "valve"=enum16{"A", "B", "ALL"}."B", "action"=T48."MOVE VALVE") -> ("error out"=w2757:errorcluster)  [unwired: 5 in, 1 out]
                  }
                  frame #3 {
                    n1752 = Wait (ms)(milliseconds to wait=1000) -> ()  [unwired: 1 out]
                  }
                  frame #4 {
                    n1753 = case shown="True" "Force FB at end of shunt?" {
                      tunnel: w2766 -> [_ w2770]
                      frame False {
                      }
                      frame True {
                        w2769 = TRUE
                        n1754 = local write "Trap Pos. FB ON"(w2769) -> ()
                        n1755 = xnode "Read/Write Control"("FPGA VI Reference In"=w2770, "Force feedback"=w2769) -> ()  [unwired: 1 in, 2 out]
                      }
                    }
                  }
                  frame #5 {
                    n1756 = local write "Shunt 2"(FALSE) -> ()
                  }
                }
              }
            }
          }
        }
      }
      event "Inject Pump 3": Value Change {
        n1757 = event-data() -> ()  [unwired: 7 out]
        n1758 = local read "Use Harvard pumps\nfor beads (else Chemyx)"() -> (w2774:bool)
        n1759 = disable-structure shown="Disabled" {
          disable-tunnel: w2774 -> [w2776 _]
          disable-tunnel: w2773 -> [w2775 _]
          frame Disabled {
            n1760 = case shown="True" w2776 {
              tunnel: "Inject Pump 3" -> [w2780 w2821]
              tunnel: w2775 -> [_ w2822]
              frame False {
                n1761 = local read "Pump write delay (ms)"() -> (w2779:dbl)
                n1762 = case shown="True" w2780 {
                  tunnel: w2779 -> [w2786 w2800]
                  tunnel: "Chemyx Syringe Pump Serial Port" -> [w2783 w2799]
                  frame False {
                    n1763 = flat-sequence {
                      tunnel: w2783 -> [w2787]
                      tunnel: [w2787] -> w2784
                      tunnel: w2786 -> [_]
                      tunnel: [w2790] -> w2785
                      tunnel: w2784 -> [w2790]
                      tunnel: w2785 -> [w2791]
                      tunnel: [w2791] -> w2781
                      tunnel: [w2793] -> w2782
                      tunnel: w2781 -> [w2793]
                      tunnel: w2782 -> [w2795]
                      frame #0 {
                        n1764 = call "Write to pump.vi"("string"="enter pump3", "VISA resource name"=w2787) -> ()  [unwired: 1 out]
                      }
                      frame #1 {
                        n1765 = local read "Pump pause delay (ms)"() -> (w2789:u32)
                        n1766 = Wait (ms)(milliseconds to wait=w2789) -> ()  [unwired: 1 out]
                      }
                      frame #2 {
                        n1767 = call "Write to pump.vi"("string"="stop", "VISA resource name"=w2791) -> ()  [unwired: 1 out]
                      }
                      frame #3 {
                        n1768 = Wait (ms)(milliseconds to wait=u32 0) -> ()  [unwired: 1 out]
                      }
                      frame #4 {
                        n1769 = call "Write to pump.vi"("string"="stop", "VISA resource name"=w2795) -> ()  [unwired: 1 out]
                      }
                    }
                  }
                  frame True {
                    n1770 = flat-sequence {
                      tunnel: w2799 -> [w2809]
                      tunnel: w2800 -> [w2804]
                      tunnel: w2800 -> [w2811]
                      tunnel: w2799 -> [w2812]
                      tunnel: [w2812] -> w2798
                      tunnel: [w2815] -> w2797
                      tunnel: w2798 -> [w2815]
                      tunnel: w2797 -> [w2816]
                      frame #0 {
                        n1771 = local read "All Pump Parameters"() -> (w2803:T14)
                        n1772 = Unbundle By Name(w2803) -> ("Pump 3"=w2810:T57)
                        n1773 = call "Set pump parameters.vi"("Pump write delay (ms)"=w2804, "Volume (uL)"="Ch 3 Inject Volume (uL)", "Rate (uL/h)"="Ch 3 Inject Rate (ul/h)", "Units"=4.0, "Pump #"=3.0, "Pump Parameters In"=w2810, "VISA resource name"=w2809) -> ("Pump Parameters Out"=w2802:T57)  [unwired: 3 in]
                        n1774 = Bundle By Name(cluster=w2803, "Pump 3"=w2802) -> (w2801:T14)
                        n1775 = local write "All Pump Parameters"(w2801) -> ()
                      }
                      frame #1 {
                        n1776 = Wait (ms)(milliseconds to wait=w2811) -> ()  [unwired: 1 out]
                      }
                      frame #2 {
                        n1777 = call "Write to pump.vi"("string"="start", "VISA resource name"=w2812) -> ()  [unwired: 1 out]
                      }
                      frame #3 {
                        n1778 = Wait (ms)(milliseconds to wait=u32 500) -> ()  [unwired: 1 out]
                      }
                      frame #4 {
                        n1779 = call "Write to pump.vi"("string"="start", "VISA resource name"=w2816) -> ()  [unwired: 1 out]
                      }
                    }
                  }
                }
              }
              frame True {
                n1780 = case shown="False" w2821 {
                  tunnel: w2822 -> [w2834 w2841]
                  frame False {
                    n1781 = flat-sequence {
                      tunnel: w2834 -> [w2836]
                      frame #0 {
                        n1782 = local write "Flushing P3"(FALSE ("Flushing P3")) -> ()
                        n1783 = Concatenate Strings("stop" ("string"), "\r") -> (w2838:string)
                        n1784 = VISA Write(VISA resource name=w2836, write buffer=w2838) -> ()  [unwired: 1 in, 3 out]
                      }
                      frame #1 {
                        n1785 = property on="Clear Volume P3" class="Bool (strict)"("Val(Sgnl)"=TRUE ("Value (Signaling)")) -> ()  [unwired: 2 in, 2 out]
                      }
                    }
                  }
                  frame True {
                    n1786 = local read "Normal Flow Rate (ul/h) P3"() -> (w2842:dbl)
                    n1787 = Number To Decimal String(number=w2842) -> (decimal integer string=w2848:string)  [unwired: 1 in]
                    n1788 = Concatenate Strings("irate  " ("string"), w2848, " u/h" ("string"), "\r") -> (w2846:string)
                    n1789 = VISA Write(VISA resource name=w2841, write buffer=w2846) -> (VISA resource name out=w2844:refnum<visa-resource-name>)  [unwired: 1 in, 2 out]
                    n1790 = Concatenate Strings("irun" ("string"), "\r") -> (w2850:string)
                    n1791 = VISA Write(VISA resource name=w2844, write buffer=w2850) -> ()  [unwired: 1 in, 3 out]
                  }
                }
                n1792 = local read "Save Event Log?"() -> (w2819:bool)
                n1793 = local read "Saving..."() -> (w2820:bool)
                n1794 = And(x=w2820, y=w2819) -> (x .and. y?=w2818:bool)
                n1795 = case shown="True" w2818 {
                  tunnel: w2821 -> [_ w2829]
                  frame False {
                  }
                  frame True {
                    n1796 = local read "Normal Flow Rate (ul/h) P3"() -> (w2823:dbl)
                    n1797 = Number To Decimal String(number=w2823) -> (decimal integer string=w2825:string)  [unwired: 1 in]
                    n1798 = Concatenate Strings("on, flow rate", w2825) -> (w2824:string)
                    n1799 = local read "log file ref"() -> (w2828:refnum<file>)
                    n1800 = Select(t=w2824, s=w2829, f="off") -> (s? t:f=w2830:string)
                    n1801 = local read "Time (s)"() -> (w2827:dbl)
                    n1802 = Concatenate Strings("pump 3 ", w2830) -> (w2832:string)
                    n1803 = call "write to event log.vi"("log file ref"=w2828, "time"=w2827, "input string"=w2832) -> ()  [unwired: 8 in]
                  }
                }
              }
            }
          }
          frame Enabled {
          }
        }
      }
      event "Inject Pump 2": Value Change {
        n1804 = event-data() -> ()  [unwired: 7 out]
        n1805 = local read "Pump write delay (ms)"() -> (w2857:dbl)
        n1806 = local read "Chemyx Syringe Pump Serial Port"() -> (w2856:refnum<visa-resource-name>)
        n1807 = flat-sequence {
          tunnel: w2856 -> [w2881]
          tunnel: w2857 -> [w2877]
          tunnel: "Inject Pump 2" -> [_]
          tunnel: w2857 -> [w2883]
          tunnel: w2856 -> [w2884]
          frame #0 {
            n1808 = local read "All Pump Parameters"() -> (w2876:T14)
            n1809 = Multiply(x=60.0, y="Flush Center Ch Rate (ul/m)") -> (x*y=w2873:dbl)
            n1810 = Unbundle By Name(w2876) -> ("Pump 2"=w2882:T57)
            n1811 = call "Set pump parameters.vi"("Pump write delay (ms)"=w2877, "Volume (uL)"="Flush Center Ch Volume (uL)", "Rate (uL/h)"=w2873, "Units"=3.0, "Pump #"=2.0, "Pump Parameters In"=w2882, "VISA resource name"=w2881) -> ("Pump Parameters Out"=w2875:T57)  [unwired: 3 in]
            n1812 = Bundle By Name(cluster=w2876, "Pump 2"=w2875) -> (w2874:T14)
            n1813 = local write "All Pump Parameters"(w2874) -> ()
            n1814 = Add(x="Flush Center Ch Volume (uL)", y="Total Volume\nFlushed (uL)") -> (x+y=w2870:dbl)
            n1815 = local write "Total Volume\nFlushed (uL)"(w2870) -> ()
          }
          frame #1 {
            n1816 = Wait (ms)(milliseconds to wait=w2883) -> ()  [unwired: 1 out]
          }
          frame #2 {
            n1817 = call "Write to pump.vi"("string"="start", "VISA resource name"=w2884) -> ()  [unwired: 1 out]
          }
        }
        n1818 = local read "Save Event Log?"() -> (w2855:bool)
        n1819 = local read "Saving..."() -> (w2854:bool)
        n1820 = And(x=w2855, y=w2854) -> (x .and. y?=w2853:bool)
        n1821 = case shown="True" w2853 {
          tunnel: "Inject Pump 2" -> [_ w2864]
          frame False {
          }
          frame True {
            n1822 = local read "Flow rate (uL/h)"() -> (w2858:dbl)
            n1823 = Number To Decimal String(number=w2858) -> (decimal integer string=w2860:string)  [unwired: 1 in]
            n1824 = Concatenate Strings("on, flow rate", w2860) -> (w2859:string)
            n1825 = Select(t=w2859, s=w2864, f="off") -> (s? t:f=w2868:string)
            n1826 = local read "Time (s)"() -> (w2862:dbl)
            n1827 = local read "log file ref"() -> (w2863:refnum<file>)
            n1828 = Concatenate Strings("pump 2 ", w2868) -> (w2866:string)
            n1829 = call "write to event log.vi"("log file ref"=w2863, "time"=w2862, "input string"=w2866) -> ()  [unwired: 8 in]
          }
        }
      }
      event "Sample Channel\nFlow": Value Change {
        n1830 = event-data() -> ()  [unwired: 7 out]
        n1831 = disable-structure shown="Disabled" {
          disable-tunnel: w2886 -> [w2893 _]
          frame Disabled {
            n1832 = Select(t="irun" ("string"), s="Sample Channel\nFlow", f="stop" ("string")) -> (s? t:f=w2888:string)
            n1833 = Concatenate Strings(w2888, "\r") -> (w2891:string)
            n1834 = VISA Write(VISA resource name=w2893, write buffer=w2891) -> ()  [unwired: 1 in, 3 out]
          }
          frame Enabled {
          }
        }
      }
      event "Start Flow": Value Change {
        n1835 = event-data() -> ()  [unwired: 7 out]
        n1836 = disable-structure shown="Disabled" {
          disable-tunnel: w2894 -> [w2895 _]
          frame Disabled {
            n1837 = local write "Sample Channel\nFlow"(TRUE ("Sample Channel\nFlow")) -> ()
            n1838 = local write "Start Flow"(FALSE ("Start Flow")) -> ()
            n1839 = Concatenate Strings("irun" ("string"), "\r") -> (w2899:string)
            n1840 = VISA Write(VISA resource name=w2895, write buffer=w2899) -> ()  [unwired: 1 in, 3 out]
          }
          frame Enabled {
          }
        }
      }
      event "Stop Flow": Value Change {
        n1841 = event-data() -> ()  [unwired: 7 out]
        n1842 = disable-structure shown="Disabled" {
          disable-tunnel: w2901 -> [w2903 _]